vi "UHR-Fleezers Control (host) - 12.0.vi"() -> ()   [LabVIEW 2014] (continued)
        n1715 = call "Update messages.vi"("Message to add"=w2420, "Old message string"=w2425) -> ("New message string"=w2419:string)
        n1716 = local write "Messages"(w2419) -> ()
      }
      event "Load user params": Value Change {
        n1717 = event-data() -> ()  [unwired: 7 out]
        n1718 = local write "Load user params"(FALSE ("Read user\nparams")) -> ()
        n1719 = flat-sequence {
          tunnel: [w2457] -> w2445
          tunnel: [w2456] -> w2443
          tunnel: [w2455] -> w2441
          tunnel: [w2454] -> w2439
          tunnel: [w2453] -> w2437
          tunnel: [w2452] -> w2435
          tunnel: [w2451] -> w2433
          tunnel: [w2450] -> w2431
          tunnel: [w2449] -> w2429
          tunnel: [w2448] -> w2427
          tunnel: [w2467] -> w2446
          tunnel: w2445 -> [w2467]
          tunnel: [w2466] -> w2444
          tunnel: w2443 -> [w2466]
          tunnel: [w2465] -> w2442
          tunnel: w2441 -> [w2465]
          tunnel: [w2464] -> w2440
          tunnel: w2439 -> [w2464]
          tunnel: [w2463] -> w2438
          tunnel: w2437 -> [w2463]
          tunnel: [w2462] -> w2436
          tunnel: w2435 -> [w2462]
          tunnel: [w2461] -> w2434
          tunnel: w2433 -> [w2461]
          tunnel: [w2460] -> w2432
          tunnel: w2431 -> [w2460]
          tunnel: [w2459] -> w2430
          tunnel: w2429 -> [w2459]
          tunnel: [w2458] -> w2428
          tunnel: w2427 -> [w2458]
          tunnel: w2446 -> [w2484]
          tunnel: w2444 -> [w2483]
          tunnel: w2442 -> [w2482]
          tunnel: w2440 -> [w2481]
          tunnel: w2438 -> [w2480]
          tunnel: w2436 -> [w2479]
          tunnel: w2434 -> [w2478]
          tunnel: w2432 -> [w2477]
          tunnel: w2430 -> [w2476]
          tunnel: w2428 -> [w2475]
          frame #0 {
            # "Make exceptions.\nThese will not be\nloaded."
            n1720 = local read "Sample Channel\nFlow"() -> (w2452:bool)
            n1721 = local read "Green ON/Interlacing"() -> (w2453:bool)
            n1722 = local read "Trap 1 (ON/OFF)"() -> (w2457:bool)
            n1723 = local read "Trap 2 (ON/OFF)"() -> (w2456:bool)
            n1724 = local read "Trap Pos. FB ON"() -> (w2448:bool)
            n1725 = local read "Inject Pump 1"() -> (w2451:bool)
            n1726 = local read "Inject Pump 3"() -> (w2450:bool)
            n1727 = local read "Trap D (MHz)"() -> (w2449:dbl)
            n1728 = local read "Index"() -> (w2454:dbl)
            n1729 = local read "Fish"() -> (w2455:bool)
          }
          frame #1 {
            n1730 = local read "User"() -> (w2468:string)
            n1731 = call "retrieve control values.vi"("User"=w2468) -> ()  [unwired: 10 in, 1 out]
            n1732 = local read "Messages"() -> (w2474:string)
            n1733 = Concatenate Strings("User: ", w2468, "\r", "Parameters loaded.") -> (w2469:string)
            n1734 = call "Update messages.vi"("Message to add"=w2469, "Old message string"=w2474) -> ("New message string"=w2473:string)
            n1735 = local write "Messages"(w2473) -> ()
          }
          frame #2 {
            n1736 = local write "Sample Channel\nFlow"(w2479) -> ()
            n1737 = local write "Green ON/Interlacing"(w2480) -> ()
            n1738 = local write "Trap 1 (ON/OFF)"(w2484) -> ()
            n1739 = local write "Trap 2 (ON/OFF)"(w2483) -> ()
            n1740 = local write "Inject Pump 1"(w2478) -> ()
            n1741 = local write "Trap Pos. FB ON"(w2475) -> ()
            n1742 = local write "Inject Pump 3"(w2477) -> ()
            n1743 = local write "Trap D (MHz)"(w2476) -> ()
            n1744 = local write "Index"(w2481) -> ()
            n1745 = local write "Fish"(w2482) -> ()
          }
        }
      }
      event "Abort wiggle": Value Change {
        n1746 = event-data() -> ()  [unwired: 7 out]
        n1747 = flat-sequence {
          tunnel: w2488 -> [w2492]
          tunnel: w2487 -> [w2491]
          tunnel: [w2490] -> w2485
          tunnel: [w2494] -> w2486
          tunnel: w2485 -> [w2494]
          frame #0 {
            n1748 = xnode "Read/Write Control"("FPGA VI Reference In"=w2492, "error in"=w2491, "Abort wiggle 1"="Abort wiggle", "Abort wiggle 2"="Abort wiggle") -> ("error out"=w2490:errorcluster)  [unwired: 1 out]
          }
          frame #1 {
            n1749 = local write "Abort wiggle"(FALSE ("Abort wiggle")) -> ()
          }
        }
      }
    }
    "error out 2" <- w1265
    n1750 = node-c288() -> ()  [unwired: 2 out]
  }
  n1751 = node-c288() -> (w126:T26)  [unwired: 4 in]
  n1752 = local write "Target size"(cluster{"Width":dbl, "Height":dbl} {"Width"=40.0, "Height"=40.0} ("Target size")) -> ()
  n1753 = timed-loop "Run Scripts, including: stage motion" {
    tunnel: w130 -> [w2502]
    tunnel: w5 -> [w2503]
    tunnel: [w2503] -> w129
    tunnel: [w2502] -> w128
    timing: w126 -> [_]
    timing-out: [_] -> w125
    tunnel: w111 -> [w2501]
    tunnel: w112 -> [w2500]
    tunnel: w55 -> [w2497]
    tunnel: w54 -> [w2496]
    tunnel: w53 -> [w2498]
    tunnel: w52 -> [w2499]
    stop <- w2495 stop-if-true
    n1754 = node-c288() -> ()  [unwired: 1 in, 1 out]
    n1755 = event shown="[10] \"Move to Position 1\", \"Move to Position 2\", \"Move to Position 3\", \"Move to Position 4\", \"Move to Position 5\", \"Lower Ch. Cap.\": Value Change" {
      selector: _ -> [_ _ _ _ _ _ _ _ _ _ _ _ _ _ _ _ _ _ _ _ _]
      dyn-events: _ -> [_ _ _ _ _ _ _ _ _ _ _ _ _ _ _ _ _ _ _ _ _]
      timeout: _ -> [_ _ _ _ _ _ _ _ _ _ _ _ _ _ _ _ _ _ _ _ _]
      tunnel: ["Set Position" "Move to Position" _ _ "Read Harvard" _ _ _ _ _ _ _ "Got ADig bead" "Force FB Script" "Rupture Script" _ "Got DNA bead" "Take Stepping Data" _ "Take Detection Laser\nImage" _] -> _
      tunnel: [_ _ _ _ _ _ _ _ _ _ _ _ _ _ _ _ _ _ _ _ w3178] -> w2495
      tunnel: w2502 -> [w2521 w2529 w2542 w2572 _ w2620 w2660 w2743 w2774 w2908 w2936 w2971 _ w2989 _ _ _ _ _ _ _]
      tunnel: w2503 -> [w2522 w2530 w2543 w2573 _ w2621 w2661 w2744 w2775 w2909 w2937 w2972 _ w2990 _ _ _ _ _ _ _]
      tunnel: w2501 -> [_ _ _ _ w2605 _ _ _ _ _ _ _ _ _ _ _ _ _ _ _ _]
      tunnel: w2500 -> [_ _ _ _ w2604 _ _ _ _ _ _ _ _ _ _ _ _ _ _ _ _]
      tunnel: w2499 -> [_ _ _ _ _ _ _ _ _ _ _ _ _ _ _ _ _ _ _ _ _]
      tunnel: w2498 -> [_ _ _ _ _ _ _ _ _ _ _ _ _ _ _ _ _ _ _ _ _]
      tunnel: w2497 -> [_ _ _ _ _ _ _ _ _ _ _ _ _ _ _ _ _ _ _ _ _]
      tunnel: w2496 -> [_ _ _ _ _ _ _ _ _ _ _ _ _ _ _ _ _ _ _ _ _]
      event "Set Position", "Set Position 2", "Set Position 3", "Set Position 4", "Set Position 5", "Set Position 1": Value Change {
        n1756 = event-data() -> ()  [unwired: 1 in, 5 out]
        n1757 = Build Array("Set Position 1", "Set Position 2", "Set Position 3", "Set Position 4", "Set Position 5") -> (w2520:bool[])
        n1758 = Boolean Array To Number(Boolean array=w2520) -> (number=w2519:u32)
        n1759 = Logarithm Base 2(1:w2519) -> (0:w2511:dbl)
        n1760 = call "Read Stage Position.vi"("error in"=w2521, "VISA resource name in"=w2522) -> ("Current Position"=w2526:cluster{dbl, dbl, dbl}, "error out"=w2525:errorcluster)  [unwired: 2 out]
        n1761 = Decrement(x="Position") -> (x-1=w2509:dbl)
        n1762 = Greater Or Equal?(x=w2511, y=0.0) -> (x >= y?=w2512:bool)
        n1763 = Cluster To Array(cluster=w2526) -> (array=w2523:dbl[])
        n1764 = local write "Stage Control Serial Error"(w2525) -> ()
        n1765 = Select(t=w2511, s=w2512, f=w2509) -> (s? t:f=w2508:dbl)
        n1766 = Increment(x=w2508) -> (x+1=w2507:dbl)
        n1767 = Build Array (concatenate)(w2507, w2523) -> (w2506:dbl[])
        n1768 = Replace Array Subset(array="Saved Stage Positions", new element=w2506, index (row)=w2508) -> (w2524:dbl[][])  [unwired: 1 in]
        n1769 = local write "Saved Stage Positions"(w2524) -> ()
      }
      event "Move to Position": Value Change {
        n1770 = event-data() -> ()  [unwired: 1 in, 5 out]
        n1771 = flat-sequence {
          tunnel: w2530 -> [w2534]
          tunnel: w2529 -> [w2533]
          frame #0 {
            n1772 = local read "Saved Stage Positions"() -> (w2536:dbl[][])
            n1773 = local read "Position"() -> (w2535:dbl)
            n1774 = local write "Stage Moving"(TRUE ("Stage Moving")) -> ()
            n1775 = call "move to saved stage position.vi"("error in"=w2533, "Stage VISA resource name in"=w2534, "Position"=w2535, "Saved Stage Positions"=w2536) -> ("error out"=w2532:errorcluster)  [unwired: 1 out]
            n1776 = local write "Stage Control Serial Error"(w2532) -> ()
          }
          frame #1 {
            n1777 = call <vilib>:"Beep.vi"() -> ()  [unwired: 3 in, 9 out]
            n1778 = local write "Stage Moving"(FALSE ("Stage Moving")) -> ()
          }
        }
      }
      event "Move Cap. 1 (DNA Bottom)": Value Change {
        n1779 = event-data() -> ()  [unwired: 1 in, 5 out]
        n1780 = local write "Move Cap. 1 (DNA Bottom)"(FALSE ("Move Cap. 1 (DNA Right)")) -> ()
        n1781 = flat-sequence {
          tunnel: w2542 -> [w2545]
          tunnel: w2543 -> [w2546]
          tunnel: [w2546] -> w2540
          tunnel: [w2545] -> w2539
          tunnel: w2540 -> [w2548]
          tunnel: w2539 -> [w2547]
          frame #0 {
            n1782 = property on="Sample Channel\nFlow" class="Bool (strict)"("Val(Sgnl)"="Cap 1 Samp Flow ON") -> ()  [unwired: 2 in, 2 out]
          }
          frame #1 {
            n1783 = local read "Saved Stage Positions"() -> (w2558:dbl[][])
            n1784 = local write "Stage Moving"(TRUE ("Stage Moving")) -> ()
            n1785 = Array Subset(array=w2558, index (row)=0 ("index"), length (row)=1 ("length"), index (col)=1 ("index"), length (col)=3 ("length")) -> (w2555:dbl[][])
            n1786 = Reshape Array(w2555, 3 ("dimension size")) -> (w2553:dbl[])
            n1787 = Array To Cluster(array=w2553) -> (cluster=w2552:cluster{"[0]":dbl, "[1]":dbl, "[2]":dbl})
            n1788 = call "Set Stage Position.vi"("Position"=w2552, "error in"=w2547, "VISA resource name in"=w2548) -> ("error out"=w2551:errorcluster)  [unwired: 2 out]
            n1789 = local write "Stage Control Serial Error"(w2551) -> ()
          }
          frame #2 {
            n1790 = local write "Stage Moving"(FALSE ("Stage Moving")) -> ()
            n1791 = case shown="True" "Cap 1 Flow ON" {
              frame False {
              }
              frame True {
                n1792 = property on="Inject Pump 1" class="Bool (strict)"("Val(Sgnl)"=TRUE ("Value (Signaling)")) -> ()  [unwired: 2 in, 2 out]
              }
            }
            n1793 = call <vilib>:"Beep.vi"() -> ()  [unwired: 3 in, 9 out]
          }
          frame #3 {
            n1794 = property on="Sample Channel\nFlow" class="Bool (strict)"("Val(Sgnl)"=FALSE ("Value (Signaling)")) -> ()  [unwired: 2 in, 2 out]
            n1795 = local read "Cap. 2 BD T1?\n(ADig T1, DNA T2)"() -> (w2565:bool)
            n1796 = case shown="True" w2565 {
              tunnel: "Cap 1 T ON" -> [w2567 w2568]
              frame False {
                n1797 = property on="Trap 1 (ON/OFF)" class="Bool (strict)"("Val(Sgnl)"=w2567) -> ()  [unwired: 2 in, 2 out]
              }
              frame True {
                n1798 = property on="Trap 2 (ON/OFF)" class="Bool (strict)"("Val(Sgnl)"=w2568) -> ()  [unwired: 2 in, 2 out]
              }
            }
            n1799 = property on="Got DNA bead" class="Bool (strict)"("Key Focus"=TRUE) -> ()  [unwired: 2 in, 2 out]
          }
        }
      }
      event "Move Cap. 2 (ADig Top)": Value Change {
        n1800 = event-data() -> ()  [unwired: 1 in, 5 out]
        n1801 = local write "Move Cap. 2 (ADig Top)"(FALSE ("Move Cap. 2 (ADig Left)")) -> ()
        n1802 = flat-sequence {
          tunnel: w2572 -> [w2575]
          tunnel: w2573 -> [w2576]
          tunnel: [w2576] -> w2570
          tunnel: [w2575] -> w2569
          tunnel: w2570 -> [w2578]
          tunnel: w2569 -> [w2577]
          frame #0 {
            n1803 = property on="Sample Channel\nFlow" class="Bool (strict)"("Val(Sgnl)"="Cap 2 Samp Flow ON") -> ()  [unwired: 2 in, 2 out]
          }
          frame #1 {
            n1804 = local read "Saved Stage Positions"() -> (w2588:dbl[][])
            n1805 = local write "Stage Moving"(TRUE ("Stage Moving")) -> ()
            n1806 = Array Subset(array=w2588, index (row)=1 ("index"), length (row)=1 ("length"), index (col)=1 ("index"), length (col)=3 ("length")) -> (w2585:dbl[][])
            n1807 = disable-structure shown="Disabled" {
              frame Disabled {
                w2590 = FALSE ("Value (Signaling)")
                n1808 = property on="Trap 1 (ON/OFF)" class="Bool (strict)"("Val(Sgnl)"=w2590) -> ()  [unwired: 2 in, 2 out]
                n1809 = property on="Trap 1 (ON/OFF)" class="Bool (strict)"("Val(Sgnl)"=w2590) -> ()  [unwired: 2 in, 2 out]
              }
              frame Enabled {
              }
            }
            n1810 = Reshape Array(w2585, 3 ("dimension size")) -> (w2583:dbl[])
            n1811 = Array To Cluster(array=w2583) -> (cluster=w2582:cluster{"[0]":dbl, "[1]":dbl, "[2]":dbl})
            n1812 = call "Set Stage Position.vi"("Position"=w2582, "error in"=w2577, "VISA resource name in"=w2578) -> ("error out"=w2581:errorcluster)  [unwired: 2 out]
            n1813 = local write "Stage Control Serial Error"(w2581) -> ()
          }
          frame #2 {
            n1814 = local write "Stage Moving"(FALSE ("Stage Moving")) -> ()
            n1815 = call <vilib>:"Beep.vi"() -> ()  [unwired: 3 in, 9 out]
            n1816 = case shown="True" "Cap 2 Flow ON" {
              frame False {
              }
              frame True {
                n1817 = property on="Inject Pump 3" class="Bool (strict)"("Val(Sgnl)"=TRUE ("Value (Signaling)")) -> ()  [unwired: 2 in, 2 out]
              }
            }
          }
          frame #3 {
            n1818 = Wait (ms)(milliseconds to wait=u32 500) -> ()  [unwired: 1 out]
          }
          frame #4 {
            n1819 = local read "Cal @ (MHz)"() -> (w2596:dbl)
            n1820 = property on="Sample Channel\nFlow" class="Bool (strict)"("Val(Sgnl)"=FALSE ("Value (Signaling)")) -> ()  [unwired: 2 in, 2 out]
            n1821 = case shown="False" "Cap. 2 BD T1?\n(ADig T1, DNA T2)" {
              tunnel: "Cap 2 T ON" -> [w2601 w2602]
              frame False {
                n1822 = property on="Trap 2 (ON/OFF)" class="Bool (strict)"("Val(Sgnl)"=w2601) -> ()  [unwired: 2 in, 2 out]
              }
              frame True {
                n1823 = property on="Trap 1 (ON/OFF)" class="Bool (strict)"("Val(Sgnl)"=w2602) -> ()  [unwired: 2 in, 2 out]
              }
            }
            n1824 = property on="Got ADig bead" class="Bool (strict)"("Key Focus"=TRUE) -> ()  [unwired: 2 in, 2 out]
            n1825 = local write "Target"("Target\nON?") -> ()
            n1826 = property on="Trap D (MHz)" class="DigNum (strict)"("Val(Sgnl)"=w2596) -> ()  [unwired: 2 in, 2 out]
          }
        }
      }
      event "Read Harvard": Value Change {
        n1827 = event-data() -> ()  [unwired: 1 in, 5 out]
        n1828 = Concatenate Strings("write buffer", "\r") -> (w2607:string)
        n1829 = VISA Write(VISA resource name=w2605, write buffer=w2607, error in (no error)=w2604) -> (VISA resource name out=w2616:refnum<visa-resource-name>, error out=w2615:errorcluster)  [unwired: 1 out]
        n1830 = stacked-sequence {
          tunnel: [w2619] -> w2614
          tunnel: w2616 -> [w2619]
          tunnel: w2615 -> [w2618]
          tunnel: [w2618] -> w2609
          frame #0 {
            n1831 = Wait (ms)(milliseconds to wait=50) -> ()  [unwired: 1 out]
          }
        }
        n1832 = property class="Instr"(reference=w2614, error in=w2609) -> (reference out=w2613:refnum<visa-resource-name>, error out=w2611:errorcluster, "Serial Settings:Number of Bytes at Serial Port"=w2612:u32)
        "Serial Settings:Number of Bytes at Serial Port" <- w2612
        n1833 = VISA Read(VISA resource name=w2613, byte count=w2612, error in (no error)=w2611) -> (read buffer=w2610:string)  [unwired: 3 out]
        "read buffer" <- w2610
        n1834 = Fract/Exp String To Number(string=w2610) -> ()  [unwired: 5 out]
      }
      event "+z", "-z": Value Change {
        n1835 = event-data() -> ()  [unwired: 1 in, 5 out]
        n1836 = flat-sequence {
          tunnel: w2620 -> [w2642]
          tunnel: w2621 -> [w2622]
          frame #0 {
            n1837 = call "Read Stage Position.vi"("error in"=w2642, "VISA resource name in"=w2622) -> ("Current Position"=w2627:cluster{dbl, dbl, dbl}, "error out"=w2640:errorcluster, "VISA resource name out"=w2641:refnum<visa-resource-name>)  [unwired: 1 out]
            n1838 = local read "Saved Stage Positions"() -> (w2651:dbl[][])
            n1839 = Divide(x="z nudge increment (um)", y=1000.0) -> (x/y=w2639:dbl)
            n1840 = Boolean To (0,1)(Boolean="+z") -> (0, 1=w2631:i16)
            n1841 = Boolean To (0,1)(Boolean="-z") -> (0, 1=w2632:i16)
            n1842 = Array Subset(array=w2651, index (row)=1 ("index"), length (row)=1 ("length"), index (col)=1 ("index"), length (col)=3 ("length")) -> (w2648:dbl[][])
            n1843 = Multiply(x=w2631, y=w2639) -> (x*y=w2635:dbl)
            n1844 = Multiply(x=w2632, y=w2639) -> (x*y=w2633:dbl)
            n1845 = Unbundle(w2627) -> (w2625:dbl, w2624:dbl, w2628:dbl)
            n1846 = Negate(x=w2633) -> (-x=w2634:dbl)
            n1847 = Reshape Array(w2648, 3 ("dimension size")) -> (w2646:dbl[])
            n1848 = Add(x=w2635, y=w2634) -> (x+y=w2636:dbl)
            n1849 = Array To Cluster(array=w2646) -> ()  [unwired: 1 out]
            n1850 = Add(x=w2636, y=w2628) -> (x+y=w2626:dbl)
            n1851 = Bundle(cluster=w2627, w2625, w2624, w2626) -> (w2623:cluster{dbl, dbl, dbl})
            n1852 = call "Set Stage Position.vi"("Position"=w2623, "error in"=w2640, "VISA resource name in"=w2641) -> ("error out"=w2645:errorcluster)  [unwired: 2 out]
            n1853 = local write "Stage Moving"(TRUE ("Stage Moving")) -> ()
            n1854 = local write "Stage Control Serial Error"(w2645) -> ()
          }
          frame #1 {
            n1855 = local write "Stage Moving"(FALSE ("Stage Moving")) -> ()
            n1856 = call <vilib>:"Beep.vi"() -> ()  [unwired: 3 in, 9 out]
          }
        }
      }
      event "Cal/Data Acq. Spot": Value Change {
        n1857 = event-data() -> ()  [unwired: 1 in, 5 out]
        n1858 = flat-sequence {
          tunnel: w2660 -> [w2664]
          tunnel: w2661 -> [w2665]
          tunnel: [w2665] -> w2657
          tunnel: [w2664] -> w2656
          tunnel: w2657 -> [w2670]
          tunnel: w2656 -> [w2669]
          tunnel: ["Cal @ (MHz)"] -> w2654
          tunnel: [w2674] -> w2658
          tunnel: w2654 -> [w2674]
          tunnel: w2658 -> [w2685]
          tunnel: ["W/ Offset 1"] -> w2655
          tunnel: w2658 -> [w2706]
          tunnel: w2655 -> [w2704]
          frame #0 {
            n1859 = property on="Sample Channel\nFlow" class="Bool (strict)"("Val(Sgnl)"="Daq spot flow on") -> ()  [unwired: 2 in, 2 out]
            n1860 = Wait (ms)(milliseconds to wait=u32 250) -> ()  [unwired: 1 out]
          }
          frame #1 {
            n1861 = local read "Saved Stage Positions"() -> (w2667:dbl[][])
            n1862 = property on="Trap D (MHz)" class="DigNum (strict)"("Val(Sgnl)"="Cal @ (MHz)") -> ()  [unwired: 2 in, 2 out]
            n1863 = local write "Stage Moving"(TRUE ("Stage Moving")) -> ()
            n1864 = call "move to saved stage position.vi"("error in"=w2669, "Stage VISA resource name in"=w2670, "Position"="Cal Stage Position", "Saved Stage Positions"=w2667) -> ("error out"=w2668:errorcluster)  [unwired: 1 out]
            n1865 = local write "Stage Control Serial Error"(w2668) -> ()
          }
          frame #2 {
            n1866 = local write "Stage Moving"(FALSE ("Stage Moving")) -> ()
            n1867 = property on="Sample Channel\nFlow" class="Bool (strict)"("Val(Sgnl)"="Flow ON\nduring cal?") -> ()  [unwired: 2 in, 2 out]
            n1868 = call <vilib>:"Beep.vi"() -> ()  [unwired: 3 in, 9 out]
          }
          frame #3 {
            n1869 = local read "Wait Before Save (s)"() -> (w2677:u32)
            n1870 = Multiply(x=w2677, y=u32 1000 ("milliseconds to wait")) -> (x*y=w2678:u32)
            n1871 = Wait (ms)(milliseconds to wait=w2678) -> ()  [unwired: 1 out]
          }
          frame #4 {
            n1872 = property on="Save Calibration" class="Bool (strict)"("Val(Sgnl)"=TRUE ("Value (Signaling)")) -> ()  [unwired: 2 in, 2 out]
          }
          frame #5 {
            n1873 = Wait (ms)(milliseconds to wait=u32 2000) -> ()  [unwired: 1 out]
          }
          frame #6 {
            # "Check to see if \nsaving done"
            n1874 = while {
              stop <- w2681 stop-if-true
              n1875 = local read "Saving..."() -> (w2682:bool)
              n1876 = Wait (ms)(milliseconds to wait=u32 100) -> ()  [unwired: 1 out]
              n1877 = Not(x=w2682) -> (.not. x?=w2681:bool)
            }
          }
          frame #7 {
            n1878 = case shown="True" "W/ Offset 1" {
              tunnel: w2685 -> [_ w2686]
              frame False {
              }
              frame True {
                n1879 = stacked-sequence {
                  tunnel: w2686 -> [_ _ _ _ _ _ _ w2703]
                  frame #0 {
                    n1880 = property on="Trap D (MHz)" class="DigNum (strict)"("Val(Sgnl)"="Offset 1 Start (MHz)") -> ()  [unwired: 2 in, 2 out]
                    n1881 = Replace Array Subset(array=u32[] [0] ("Index Values"), new element="Offset 1 Set", index=0) -> (w2687:u32[])
                    n1882 = property on="Saved AOD Raster Scan Parameter Sets" class="Arr (strict)"("Index Values"=w2687) -> ()  [unwired: 2 in, 2 out]
                  }
                  frame #1 {
                    n1883 = Wait (ms)(milliseconds to wait=u32 200) -> ()  [unwired: 1 out]
                  }
                  frame #2 {
                    n1884 = property on="Load parameters" class="Bool (strict)"("Val(Sgnl)"=TRUE ("Value (Signaling)")) -> ()  [unwired: 2 in, 2 out]
                  }
                  frame #3 {
                    n1885 = Wait (ms)(milliseconds to wait=u32 200) -> ()  [unwired: 1 out]
                  }
                  frame #4 {
                    n1886 = property on="Trap Raster Scan" class="Bool (strict)"("Val(Sgnl)"=TRUE ("Value (Signaling)")) -> ()  [unwired: 2 in, 2 out]
                  }
                  frame #5 {
                    n1887 = Wait (ms)(milliseconds to wait=u32 2000) -> ()  [unwired: 1 out]
                  }
                  frame #6 {
                    n1888 = while {
                      stop <- w2700 stop-if-true
                      n1889 = local read "Raster Scanning..."() -> (w2702:bool)
                      n1890 = local read "Saving..."() -> (w2698:bool)
                      n1891 = Wait (ms)(milliseconds to wait=u32 100) -> ()  [unwired: 1 out]
                      n1892 = Not(x=w2698) -> (.not. x?=w2697:bool)
                      n1893 = Not(x=w2702) -> (.not. x?=w2699:bool)
                      n1894 = And(x=w2699, y=w2697) -> (x .and. y?=w2700:bool)
                    }
                  }
                  frame #7 {
                    n1895 = property on="Trap D (MHz)" class="DigNum (strict)"("Val(Sgnl)"=w2703) -> ()  [unwired: 2 in, 2 out]
                  }
                }
              }
            }
          }
          frame #8 {
            n1896 = local read "Save ave N"() -> (w2705:dbl)
            n1897 = case shown="False" "W/ Offset 2" {
              tunnel: w2706 -> [_ w2713]
              tunnel: w2705 -> [_ w2712]
              tunnel: w2704 -> [w2708 _]
              frame False {
                n1898 = case shown="False" w2708 {
                  frame False {
                    n1899 = Multiply(x="Cal read wait (s)", y=u32 1000 ("milliseconds to wait")) -> (x*y=w2710:u32)
                    n1900 = Wait (ms)(milliseconds to wait=w2710) -> ()  [unwired: 1 out]
                  }
                  frame True {
                  }
                }
              }
              frame True {
                n1901 = stacked-sequence {
                  tunnel: w2713 -> [_ _ _ _ _ _ _ _ _ w2734 _ _]
                  tunnel: w2712 -> [_ _ _ _ _ _ _ _ _ w2732 _ _]
                  frame #0 {
                    n1902 = property on="Save ave N" class="DigNum (strict)"("Val(Sgnl)"=1.0 ("Value (Signaling)")) -> ()  [unwired: 2 in, 2 out]
                  }
                  frame #1 {
                    n1903 = Wait (ms)(milliseconds to wait=u32 500) -> ()  [unwired: 1 out]
                  }
                  frame #2 {
                    n1904 = property on="Trap D (MHz)" class="DigNum (strict)"("Val(Sgnl)"="Offset 2 Start (MHz)") -> ()  [unwired: 2 in, 2 out]
                    n1905 = Replace Array Subset(array=u32[] [0] ("Index Values"), new element="Offset 2 Set", index=0) -> (w2718:u32[])
                    n1906 = property on="Saved AOD Raster Scan Parameter Sets" class="Arr (strict)"("Index Values"=w2718) -> ()  [unwired: 2 in, 2 out]
                  }
                  frame #3 {
                    n1907 = Wait (ms)(milliseconds to wait=u32 500) -> ()  [unwired: 1 out]
                  }
                  frame #4 {
                    n1908 = property on="Load parameters" class="Bool (strict)"("Val(Sgnl)"=TRUE ("Value (Signaling)")) -> ()  [unwired: 2 in, 2 out]
                  }
                  frame #5 {
                    n1909 = Wait (ms)(milliseconds to wait=u32 500) -> ()  [unwired: 1 out]
                  }
                  frame #6 {
                    n1910 = property on="Trap Raster Scan" class="Bool (strict)"("Val(Sgnl)"=TRUE ("Value (Signaling)")) -> ()  [unwired: 2 in, 2 out]
                  }
                  frame #7 {
                    n1911 = Wait (ms)(milliseconds to wait=u32 2000) -> ()  [unwired: 1 out]
                  }
                  frame #8 {
                    n1912 = while {
                      stop <- w2727 stop-if-true
                      n1913 = local read "Raster Scanning..."() -> (w2730:bool)
                      n1914 = local read "Saving..."() -> (w2728:bool)
                      n1915 = Wait (ms)(milliseconds to wait=u32 100) -> ()  [unwired: 1 out]
                      n1916 = Not(x=w2728) -> (.not. x?=w2726:bool)
                      n1917 = Not(x=w2730) -> (.not. x?=w2729:bool)
                      n1918 = And(x=w2729, y=w2726) -> (x .and. y?=w2727:bool)
                    }
                  }
                  frame #9 {
                    n1919 = property on="Trap D (MHz)" class="DigNum (strict)"("Val(Sgnl)"=w2734) -> ()  [unwired: 2 in, 2 out]
                    n1920 = property on="Saved AOD Raster Scan Parameter Sets" class="Arr (strict)"("Index Values"=u32[] [0]) -> ()  [unwired: 2 in, 2 out]
                    n1921 = property on="Save ave N" class="DigNum (strict)"("Val(Sgnl)"=w2732) -> ()  [unwired: 2 in, 2 out]
                  }
                  frame #10 {
                    n1922 = Wait (ms)(milliseconds to wait=u32 500) -> ()  [unwired: 1 out]
                  }
                  frame #11 {
                    n1923 = property on="Load parameters" class="Bool (strict)"("Val(Sgnl)"=TRUE ("Value (Signaling)")) -> ()  [unwired: 2 in, 2 out]
                  }
                }
              }
            }
          }
          frame #9 {
            n1924 = property on="Read Cal" class="Bool (strict)"("Val(Sgnl)"=TRUE ("Value (Signaling)")) -> ()  [unwired: 2 in, 2 out]
          }
          frame #10 {
            n1925 = Wait (ms)(milliseconds to wait=u32 1000) -> ()  [unwired: 1 out]
          }
          frame #11 {
            n1926 = property on="Fish" class="Bool (strict)"("Val(Sgnl)"=TRUE ("Value (Signaling)")) -> ()  [unwired: 2 in, 2 out]
          }
        }
        n1927 = local write "Cal/Data Acq. Spot"(FALSE ("Cal/Data Acq. Spot")) -> ()
      }
      event "Dump Beads": Value Change {
        n1928 = event-data() -> ()  [unwired: 1 in, 5 out]
        n1929 = flat-sequence {
          tunnel: ["Dump spot flow on?"] -> w2740
          tunnel: [w2752] -> w2741
          tunnel: w2740 -> [w2752]
          tunnel: w2744 -> [w2757]
          tunnel: w2743 -> [w2756]
          tunnel: [w2754] -> w2742
          tunnel: w2741 -> [w2754]
          tunnel: w2742 -> [w2768]
          frame #0 {
            w2745 = FALSE ("Value (Signaling)")
            n1930 = local read "Saving..."() -> (w2747:bool)
            n1931 = local write "Dump Beads"(FALSE ("Dump Beads")) -> ()
            n1932 = property on="Inject Pump 3" class="Bool (strict)"("Val(Sgnl)"=w2745) -> ()  [unwired: 2 in, 2 out]
            n1933 = property on="Inject Pump 1" class="Bool (strict)"("Val(Sgnl)"=w2745) -> ()  [unwired: 2 in, 2 out]
            n1934 = local write "Stop Saving"(w2747) -> ()
            n1935 = local write "Fish"(w2745) -> ()
          }
          frame #1 {
            w2748 = TRUE
            w2749 = FALSE ("Fl. Triggered...")
            n1936 = case shown="True" "Dump spot flow on?" {
              frame False {
              }
              frame True {
                n1937 = property on="Sample Channel\nFlow" class="Bool (strict)"("Val(Sgnl)"=TRUE ("Stage Moving")) -> ()  [unwired: 2 in, 2 out]
              }
            }
            n1938 = local write "Fl. Triggered..."(w2749) -> ()
            n1939 = local write "Tether"(w2749) -> ()
            n1940 = local write "Multiple tether"(w2749) -> ()
            n1941 = local write "Good tether"(w2749) -> ()
            n1942 = property on="Green ON/Interlacing" class="Bool (strict)"("Val(Sgnl)"=w2749) -> ()  [unwired: 2 in, 2 out]
            n1943 = property on="Trap Pos. FB ON" class="Bool (strict)"("Val(Sgnl)"=w2749) -> ()  [unwired: 2 in, 2 out]
            n1944 = property on="Trap Trig. Fl." class="Bool (strict)"("Val(Sgnl)"=w2749) -> ()  [unwired: 2 in, 2 out]
            n1945 = local write "Bad fit"(w2749) -> ()
            n1946 = local write "Hysteresis"(w2749) -> ()
            n1947 = property on="Fl. Triggered..." class="Bool (strict)"("Val(Sgnl)"=w2749) -> ()  [unwired: 2 in, 2 out]
            n1948 = local write "Restart DMA? (AOD)"(w2748) -> ()
            n1949 = local write "Save scans"(w2748) -> ()
            n1950 = property on="Dip for Protein" class="Bool (strict)"("Val(Sgnl)"=w2749) -> ()  [unwired: 2 in, 2 out]
            n1951 = property on="Pause dwell" class="Bool (strict)"("Val(Sgnl)"=w2749) -> ()  [unwired: 2 in, 2 out]
          }
          frame #2 {
            n1952 = property on="Trap Pos. FB Offset Factor" class="DigNum (strict)"("Val(Sgnl)"=i64 0 ("Value (Signaling)")) -> ()  [unwired: 2 in, 2 out]
          }
          frame #3 {
            n1953 = local read "Saved Stage Positions"() -> (w2758:dbl[][])
            n1954 = Array Subset(array=w2758, index (row)=3 ("index"), length (row)=1 ("length"), index (col)=1 ("index"), length (col)=3 ("length")) -> (w2763:dbl[][])
            n1955 = local write "Stage Moving"(TRUE ("Stage Moving")) -> ()
            n1956 = Reshape Array(w2763, 3 ("dimension size")) -> (w2761:dbl[])
            n1957 = Array To Cluster(array=w2761) -> (cluster=w2760:cluster{"[0]":dbl, "[1]":dbl, "[2]":dbl})
            n1958 = call "Set Stage Position.vi"("Position"=w2760, "error in"=w2756, "VISA resource name in"=w2757) -> ()  [unwired: 3 out]
          }
          frame #4 {
            w2769 = FALSE ("Value (Signaling)")
            n1959 = case shown="True" w2768 {
              frame False {
              }
              frame True {
                n1960 = property on="Sample Channel\nFlow" class="Bool (strict)"("Val(Sgnl)"=FALSE ("Stage Moving")) -> ()  [unwired: 2 in, 2 out]
              }
            }
            n1961 = property on="Trap 1 (ON/OFF)" class="Bool (strict)"("Val(Sgnl)"=w2769) -> ()  [unwired: 2 in, 2 out]
            n1962 = property on="Trap 2 (ON/OFF)" class="Bool (strict)"("Val(Sgnl)"=w2769) -> ()  [unwired: 2 in, 2 out]
            n1963 = call <vilib>:"Beep.vi"() -> ()  [unwired: 3 in, 9 out]
            n1964 = local write "Fish"(FALSE ("Fish for Tether")) -> ()
          }
          frame #5 {
            n1965 = property on="Move Cap. 2 (ADig Top)" class="Bool (strict)"("Val(Sgnl)"=TRUE ("Value (Signaling)")) -> ()  [unwired: 2 in, 2 out]
            n1966 = property on="Tab Control" class="TabCtl (strict)"("Val(Sgnl)"=T34."Status" ("Value (Signaling)")) -> ()  [unwired: 2 in, 2 out]
          }
        }
      }
      event "Dip for Protein": Value Change {
        n1967 = event-data() -> ()  [unwired: 1 in, 5 out]
        n1968 = case shown="True" "Dip for Protein" {
          tunnel: w2775 -> [_ w2777]
          tunnel: w2774 -> [_ w2776]
          frame False {
          }
          frame True {
            n1969 = while {
              tunnel: w2777 -> [w2788]
              tunnel: w2776 -> [w2787]
              i -> [w2783]
              stop <- w2778 stop-if-true
              n1970 = Increment(x=w2783) -> (x+1=→"Dip #":i32)
              n1971 = flat-sequence {
                tunnel: w2787 -> [w2799]
                tunnel: w2788 -> [w2800]
                tunnel: [w2800] -> w2792
                tunnel: [w2799] -> w2791
                tunnel: [w2793] -> w2779
                tunnel: [w2805] -> w2786
                tunnel: [w2806] -> w2785
                tunnel: w2792 -> [w2807]
                tunnel: w2791 -> [w2808]
                tunnel: [w2803] -> w2780
                tunnel: w2779 -> [w2803]
                tunnel: [w2816] -> w2790
                tunnel: w2786 -> [w2816]
                tunnel: [w2815] -> w2789
                tunnel: w2785 -> [w2815]
                tunnel: [w2812] -> w2784
                tunnel: [w2811] -> w2781
                tunnel: w2780 -> [w2811]
                tunnel: w2789 -> [w2836]
                tunnel: w2790 -> [w2837]
                tunnel: w2784 -> [w2838]
                tunnel: w2781 -> [w2835]
                tunnel: [w2897] -> w2778
                frame #0 {
                  n1972 = local read "Trap Pos. FB ON"() -> (w2793:bool)
                  n1973 = Compound Arithmetic op=AND("Flow ON\nduring dip?", "FB OFF when \nflow ON", w2793) -> (w2794:bool)
                  n1974 = case shown="True" "Move trap \nbefore dip move?" {
                    frame False {
                    }
                    frame True {
                      n1975 = property on="Trap D (MHz)" class="DigNum (strict)"("Val(Sgnl)"="Dipping D (MHz)") -> ()  [unwired: 2 in, 2 out]
                    }
                  }
                  n1976 = property on="Green ON/Interlacing" class="Bool (strict)"("Val(Sgnl)"="Green ON\nbefore dip?") -> ()  [unwired: 2 in, 2 out]
                  n1977 = property on="Sample Channel\nFlow" class="Bool (strict)"("Val(Sgnl)"="Flow ON\nduring dip?") -> ()  [unwired: 2 in, 2 out]
                  n1978 = case shown="True" w2794 {
                    frame False {
                    }
                    frame True {
                      n1979 = property on="Trap Pos. FB ON" class="Bool (strict)"("Val(Sgnl)"=FALSE ("Value (Signaling)")) -> ()  [unwired: 2 in, 2 out]
                    }
                  }
                }
                frame #1 {
                  n1980 = local read "Saved Stage Positions"() -> (w2810:dbl[][])
                  n1981 = local write "Cancel dwell"(FALSE ("Cancel dwell")) -> ()
                  n1982 = call "move to saved stage position.vi"("error in"=w2808, "Stage VISA resource name in"=w2807, "Position"="Dip Stage \nPosition", "Saved Stage Positions"=w2810) -> ("VISA resource name out"=w2805:refnum<visa-resource-name>, "error out"=w2806:errorcluster)
                }
                frame #2 {
                  n1983 = node-c288() -> (w2814:T26)  [unwired: 4 in]
                  n1984 = timed-loop {
                    timing: w2814 -> [_]
                    timing-out: [_] -> w2813
                    tunnel: [w2820] -> w2812
                    i -> [w2817]
                    stop <- w2821 stop-if-true
                    n1985 = node-c288() -> ()  [unwired: 1 in, 1 out]
                    n1986 = Greater Or Equal?(x=w2817, y="Dip Duration (s)") -> (x >= y?=w2829:bool)
                    n1987 = local read "Dip for Protein"() -> (w2822:bool)
                    n1988 = local read "Dump Beads"() -> (w2819:bool)
                    n1989 = local read "Cancel dwell"() -> (w2828:bool)
                    n1990 = local read "Pause dwell"() -> (w2825:bool)
                    n1991 = Not(x=w2822) -> (.not. x?=w2827:bool)
                    n1992 = Compound Arithmetic op=OR(w2828, w2829, w2827) -> (w2826:bool)
                    n1993 = Select(t=FALSE, s=w2825, f=w2826) -> (s? t:f=w2823:bool)
                    n1994 = Not(x=w2819) -> (.not. x?=w2818:bool)
                    n1995 = node-c288() -> ()  [unwired: 1 in, 1 out]
                    n1996 = And(x=w2822, y=w2818) -> (x .and. y?=w2820:bool)
                    n1997 = Or(x=w2823, y=w2819) -> (x .or. y?=w2821:bool)
                    "Dip Time (s)" <- w2817
                  }
                  n1998 = node-c288(w2813) -> ()  [unwired: 1 out]
                }
                frame #3 {
                  n1999 = case shown="True" w2838 {
                    tunnel: w2837 -> [_ w2843]
                    tunnel: w2836 -> [_ w2842]
                    tunnel: w2835 -> [_ w2839]
                    frame False {
                    }
                    frame True {
                      n2000 = flat-sequence {
                        tunnel: w2842 -> [w2847]
                        tunnel: w2843 -> [w2848]
                        tunnel: [w2848] -> w2841
                        tunnel: [w2847] -> w2840
                        tunnel: w2839 -> [w2844]
                        tunnel: w2841 -> [w2858]
                        tunnel: w2840 -> [w2857]
                        tunnel: w2839 -> [w2866]
                        frame #0 {
                          n2001 = local read "Sample Channel\nFlow"() -> (w2846:bool)
                          n2002 = case shown="True" w2846 {
                            tunnel: "Flow ON \nduring return\nfrom dip?" -> [w2849 w2852]
                            tunnel: w2844 -> [_ w2851]
                            frame False {
                              n2003 = case shown="True" w2849 {
                                frame False {
                                }
                                frame True {
                                n2004 = property on="Sample Channel\nFlow" class="Bool (strict)"("Val(Sgnl)"=TRUE ("Value (Signaling)")) -> ()  [unwired: 2 in, 2 out]
                                }
                              }
                            }
                            frame True {
                              n2005 = case shown="False" w2852 {
                                tunnel: w2851 -> [w2853 _]
                                frame False {
                                n2006 = property on="Trap Pos. FB ON" class="Bool (strict)"("Val(Sgnl)"=w2853) -> ()  [unwired: 2 in, 2 out]
                                n2007 = property on="Sample Channel\nFlow" class="Bool (strict)"("Val(Sgnl)"=FALSE ("Value (Signaling)")) -> ()  [unwired: 2 in, 2 out]
                                }
                                frame True {
                                }
                              }
                            }
                          }
                        }
                        frame #1 {
                          # "For turning on green laser before stage reaches lower spot"
                          n2008 = case shown="True" "Green ON\nafter start\nreturn?" {
                            frame False {
                            }
                            frame True {
                              n2009 = flat-sequence {
                                frame #0 {
                                n2010 = Multiply(x="Green delay after \nstart return (s)", y=1000.0) -> (x*y=w2863:dbl)
                                n2011 = Wait (ms)(milliseconds to wait=w2863) -> ()  [unwired: 1 out]
                                }
                                frame #1 {
                                n2012 = property on="Green ON/Interlacing" class="Bool (strict)"("Val(Sgnl)"=TRUE ("Value (Signaling)")) -> ()  [unwired: 2 in, 2 out]
                                }
                              }
                            }
                          }
                          n2013 = local read "Saved Stage Positions"() -> (w2861:dbl[][])
                          n2014 = local write "Cancel dwell"(FALSE ("Cancel dwell")) -> ()
                          n2015 = call "move to saved stage position.vi"("error in"=w2857, "Stage VISA resource name in"=w2858, "Position"="Return Stage \nPosition", "Saved Stage Positions"=w2861) -> ("error out"=w2859:errorcluster)  [unwired: 1 out]
                          n2016 = local write "Stage Control Serial Error"(w2859) -> ()
                        }
                        frame #2 {
                          n2017 = property on="Trap Pos. FB ON" class="Bool (strict)"("Val(Sgnl)"=w2866) -> ()  [unwired: 2 in, 2 out]
                          n2018 = case shown="True" "Green ON \nafter return?" {
                            frame False {
                            }
                            frame True {
                              n2019 = property on="Green ON/Interlacing" class="Bool (strict)"("Val(Sgnl)"=TRUE ("Value (Signaling)")) -> ()  [unwired: 2 in, 2 out]
                            }
                          }
                          n2020 = case shown="True" "Move trap after return?" {
                            frame False {
                            }
                            frame True {
                              n2021 = property on="Trap D (MHz)" class="DigNum (strict)"("Val(Sgnl)"="Dip Trap D 2 (MHz)") -> ()  [unwired: 2 in, 2 out]
                            }
                          }
                          n2022 = case shown="True" "Save data after return?" {
                            frame False {
                            }
                            frame True {
                              n2023 = property on="Start Saving" class="Bool (strict)"("Val(Sgnl)"=TRUE ("Value (Signaling)")) -> ()  [unwired: 2 in, 2 out]
                            }
                          }
                          n2024 = property on="Sample Channel\nFlow" class="Bool (strict)"("Val(Sgnl)"="Flow ON\nduring daq?") -> ()  [unwired: 2 in, 2 out]
                        }
                        frame #3 {
                          n2025 = node-c288() -> (w2875:T26)  [unwired: 4 in]
                          n2026 = timed-loop {
                            timing: w2875 -> [_]
                            timing-out: [_] -> w2874
                            i -> [w2876]
                            stop <- w2878 stop-if-true
                            n2027 = node-c288() -> ()  [unwired: 1 in, 1 out]
                            n2028 = local read "Dump Beads"() -> (w2877:bool)
                            n2029 = Greater Or Equal?(x=w2876, y="Dwell Duration (s)") -> (x >= y?=w2883:bool)
                            n2030 = local read "Dip for Protein"() -> (w2880:bool)
                            n2031 = Not(x=w2880) -> (.not. x?=w2879:bool)
                            n2032 = Compound Arithmetic op=OR(w2883, "Cancel dwell", w2879) -> (w2882:bool)
                            n2033 = node-c288() -> ()  [unwired: 1 in, 1 out]
                            n2034 = Select(t=FALSE, s="Pause dwell", f=w2882) -> (s? t:f=w2885:bool)
                            n2035 = Or(x=w2885, y=w2877) -> (x .or. y?=w2878:bool)
                            "Dwell Time (s)" <- w2876
                          }
                          n2036 = node-c288(w2874) -> ()  [unwired: 1 out]
                        }
                      }
                    }
                  }
                }
                frame #4 {
                  n2037 = local read "Dip for Protein"() -> (w2894:bool)
                  n2038 = local read "Tether"() -> (w2893:bool)
                  n2039 = local read "Dump Beads"() -> (w2895:bool)
                  n2040 = local write "Cancel dwell"(FALSE ("Cancel dwell")) -> ()
                  n2041 = Not(x=w2893) -> (.not. x?=w2892:bool)
                  n2042 = Not(x=w2894) -> (.not. x?=w2898:bool)
                  n2043 = Not(x="Cont. Repeat Dipping?") -> (.not. x?=w2900:bool)
                  n2044 = Compound Arithmetic op=OR(w2892, w2898, w2900, w2895) -> (w2897:bool)
                }
              }
            }
          }
        }
      }
      event "Profile": Value Change {
        n2045 = event-data() -> ()  [unwired: 1 in, 5 out]
        n2046 = flat-sequence {
          tunnel: w2909 -> [w2912]
          tunnel: w2908 -> [w2920]
          tunnel: [w2914] -> w2907
          tunnel: [w2913] -> w2906
          tunnel: [w2911] -> w2904
          tunnel: [w2910] -> w2901
          tunnel: w2907 -> [w2927]
          tunnel: w2906 -> [w2926]
          tunnel: [w2924] -> w2905
          tunnel: w2904 -> [w2925]
          tunnel: [w2923] -> w2903
          tunnel: [w2922] -> w2902
          tunnel: w2901 -> [w2922]
          tunnel: w2905 -> [w2931]
          tunnel: w2903 -> [w2930]
          tunnel: w2902 -> [w2929]
          frame #0 {
            n2047 = call "Read Stage Position.vi"("error in"=w2920, "VISA resource name in"=w2912) -> ("Current Position"=w2910:cluster{dbl, dbl, dbl}, "error out"=w2913:errorcluster, "VISA resource name out"=w2911:refnum<visa-resource-name>)  [unwired: 1 out]
            "Current Position" <- w2910
            n2048 = local write "Stage Control Serial Error"(w2913) -> ()
            n2049 = Unbundle(w2910) -> (w2917:dbl, w2919:dbl, w2915:dbl)
            n2050 = Add(x=w2919, y="Y change (mm)") -> (x+y=w2916:dbl)
            n2051 = Bundle(w2917, w2916, w2915) -> (w2914:cluster{dbl, dbl, dbl})  [unwired: 1 in]
          }
          frame #1 {
            # "move to new position and start saving"
            n2052 = local write "Stage Moving"(TRUE ("Stage Moving")) -> ()
            n2053 = local write "Start Saving"(TRUE ("Start Saving")) -> ()
            n2054 = call "Set Stage Position.vi"("Position"=w2927, "error in"=w2926, "VISA resource name in"=w2925) -> ("error out"=w2923:errorcluster, "VISA resource name out"=w2924:refnum<visa-resource-name>)  [unwired: 1 out]
          }
          frame #2 {
            # "go back to start"
            n2055 = call "Set Stage Position.vi"("Position"=w2929, "error in"=w2930, "VISA resource name in"=w2931) -> ()  [unwired: 3 out]
          }
          frame #3 {
            # "stop saving"
            n2056 = local write "Stop Saving"(TRUE ("Stop Saving")) -> ()
            n2057 = local write "Stage Moving"(FALSE ("Stage Moving")) -> ()
          }
        }
      }
      event "Move to Position 1", "Move to Position 2", "Move to Position 3", "Move to Position 4", "Move to Position 5", "Lower Ch. Cap.": Value Change {
        n2058 = event-data() -> ()  [unwired: 1 in, 5 out]
        n2059 = Or(x="Move to Position 5", y="Lower Ch. Cap.") -> (x .or. y?=w2939:bool)
        n2060 = Build Array("Move to Position 1", "Move to Position 2", "Move to Position 3", "Move to Position 4", w2939) -> (w2942:bool[])
        n2061 = Boolean Array To Number(Boolean array=w2942) -> (number=w2941:u32)
        n2062 = Logarithm Base 2(1:w2941) -> (0:w2940:dbl)
        n2063 = local write "Move to Position 2"(FALSE ("Move to Position 2")) -> ()
        n2064 = local write "Move to Position 1"(FALSE ("Move to Position 1")) -> ()
        n2065 = flat-sequence {
          tunnel: w2940 -> [w2951]
          tunnel: w2937 -> [w2949]
          tunnel: w2936 -> [w2948]
          frame #0 {
            n2066 = local read "Saved Stage Positions"() -> (w2959:dbl[][])
            n2067 = Array Subset(array=w2959, index (row)=w2951, length (row)=1 ("length"), index (col)=1 ("index"), length (col)=3 ("length")) -> (w2956:dbl[][])
            n2068 = Reshape Array(w2956, 3 ("dimension size")) -> (w2954:dbl[])
            n2069 = Array To Cluster(array=w2954) -> (cluster=w2953:cluster{"[0]":dbl, "[1]":dbl, "[2]":dbl})
            n2070 = call "Set Stage Position.vi"("Position"=w2953, "error in"=w2948, "VISA resource name in"=w2949) -> ("error out"=w2952:errorcluster)  [unwired: 2 out]
            n2071 = local write "Stage Moving"(TRUE ("Stage Moving")) -> ()
            n2072 = local write "Stage Control Serial Error"(w2952) -> ()
          }
          frame #1 {
            n2073 = local write "Stage Moving"(FALSE ("Stage Moving")) -> ()
            n2074 = call <vilib>:"Beep.vi"() -> ()  [unwired: 3 in, 9 out]
          }
        }
      }
      event "Set Current\nPos to 0,0,0": Value Change {
        # "DH is \"Define Home\""
        n2075 = event-data() -> ()  [unwired: 1 in, 6 out]
        n2076 = local write "Set Current\nPos to 0,0,0"(FALSE ("Set Current\nPos to 0,0,0")) -> ()
        n2077 = Concatenate Strings("1DH" ("string"), ";" ("string"), "2DH" ("string"), ";" ("string"), "3DH" ("string"), "\r") -> (w2967:string)
        n2078 = call-poly "VISA Configure Serial Port"("VISA resource name"=w2972, "baud rate (9600)"=u32 19200, "error in (no error)"=w2971) -> ("VISA resource name out"=w2969:refnum<visa-resource-name>, "error out"=w2968:errorcluster)  [unwired: 11 in]
        n2079 = VISA Write(VISA resource name=w2969, write buffer=w2967, error in (no error)=w2968) -> (error out=w2962:errorcluster)  [unwired: 2 out]
        n2080 = local write "Stage Control Serial Error"(w2962) -> ()
      }
      event "Got ADig bead": Value Change {
        n2081 = event-data() -> ()  [unwired: 1 in, 5 out]
        n2082 = flat-sequence {
          frame #0 {
            n2083 = local read "Cap 1 Samp Flow ON"() -> (w2978:bool)
            n2084 = case shown="True" w2978 {
              frame False {
              }
              frame True {
                n2085 = property on="Sample Channel\nFlow" class="Bool (strict)"("Val(Sgnl)"=TRUE ("Value (Signaling)")) -> ()  [unwired: 2 in, 2 out]
              }
            }
            n2086 = local write "Got ADig bead"(FALSE) -> ()
          }
          frame #1 {
            n2087 = property on="Inject Pump 3" class="Bool (strict)"("Val(Sgnl)"=FALSE ("Value (Signaling)")) -> ()  [unwired: 2 in, 2 out]
            n2088 = local write "Target"(FALSE ("Target")) -> ()
          }
          frame #2 {
            n2089 = property on="Move Cap. 1 (DNA Bottom)" class="Bool (strict)"("Val(Sgnl)"=TRUE ("Value (Signaling)")) -> ()  [unwired: 2 in, 2 out]
          }
        }
      }
      event "Force FB Script": Value Change {
        n2090 = event-data() -> ()  [unwired: 1 in, 5 out]
        n2091 = local write "Force FB Script"(FALSE ("Force FB Data\nScript")) -> ()
        n2092 = flat-sequence {
          tunnel: w2989 -> [w2993]
          tunnel: w2990 -> [w2994]
          tunnel: [w2994] -> w2985
          tunnel: [w2993] -> w2984
          tunnel: w2985 -> [w2997]
          tunnel: w2984 -> [w2996]
          tunnel: ["Trap Trig Fl."] -> w2986
          tunnel: [w3039] -> w2987
          tunnel: w2986 -> [w3039]
          tunnel: [w3043] -> w2988
          tunnel: w2987 -> [w3043]
          tunnel: w2988 -> [w3045]
          frame #0 {
            n2093 = property on="Trap D (MHz)" class="DigNum (strict)"("Val(Sgnl)"="Trap D Before Moving") -> ()  [unwired: 2 in, 2 out]
          }
          frame #1 {
            n2094 = local read "Saved Stage Positions"() -> (w2999:dbl[][])
            n2095 = local write "FB Trap Pos Offset"(0.0 ("FB Trap Pos Offset")) -> ()
            n2096 = property on="Trap Pos. FB Offset Factor" class="DigNum (strict)"("Val(Sgnl)"=i64 0 ("Value (Signaling)")) -> ()  [unwired: 2 in, 2 out]
            n2097 = local write "Stage Moving"(TRUE ("Stage Moving")) -> ()
            n2098 = call "move to saved stage position.vi"("error in"=w2996, "Stage VISA resource name in"=w2997, "Position"="Stage Position To Establish FB", "Saved Stage Positions"=w2999) -> ("error out"=w2995:errorcluster)  [unwired: 1 out]
            n2099 = local write "Stage Control Serial Error"(w2995) -> ()
          }
          frame #2 {
            n2100 = call <vilib>:"Beep.vi"("duration (msec)"=u32 100, "frequency (Hz)"=u32 20) -> ()  [unwired: 1 in, 9 out]
            n2101 = local write "Stage Moving"(FALSE ("Stage Moving")) -> ()
            n2102 = property on="Tab Control 2" class="TabCtl (strict)"("Val(Sgnl)"=T6."Feedback on Trap Position" ("Value (Signaling)")) -> ()  [unwired: 2 in, 2 out]
            n2103 = stacked-sequence {
              frame #0 {
                n2104 = Multiply(x="Wait (s)", y=u32 1000 ("milliseconds to wait")) -> (x*y=w3008:u32)
                n2105 = property on="Trap D (MHz)" class="DigNum (strict)"("Val(Sgnl)"="Starting Trap D (MHz)") -> ()  [unwired: 2 in, 2 out]
                n2106 = Wait (ms)(milliseconds to wait=w3008) -> ()  [unwired: 1 out]
              }
              frame #1 {
                n2107 = property on="Set Reading to\nSetpoint" class="Bool (strict)"("Val(Sgnl)"=TRUE ("Value (Signaling)")) -> ()  [unwired: 2 in, 2 out]
              }
            }
            n2108 = property on="Tab Control" class="TabCtl (strict)"("Val(Sgnl)"=T34."Trap Control (RF)" ("Value (Signaling)")) -> ()  [unwired: 2 in, 2 out]
          }
          frame #3 {
            n2109 = Wait (ms)(milliseconds to wait=u32 500) -> ()  [unwired: 1 out]
          }
          frame #4 {